vi "UHR-Fleezers Control (host) - 12.7d.vi"() -> ()   [LabVIEW 2012] (continued)
  T22 = cluster{"New Image":T2, "New Image":T2, "New Image":T2, "New Image":T2, "New Image":T2}
  T23 = typedef "XDNodeRunTimeDep.lvlib/timing_clust.ctl" = cluster{"Expected End [f-1]":u64, "Actual End [f-1]":u64, "Finished Late? [f-1]":bool, "Expected End [i-1]":u64, "Actual End [i-1]":u64, "Finished Late? [i-1]":bool, "Expected Start [i]":u64, "Actual Start [i]":u64, "Expected Start [f]":u64, "Actual Start [f]":u64, "Source Name":string, "Structure Name":string, "Period":i64, "Deadline":i64, "Offset":i64, "Start":i64, "Priority":i32, "Timeout":i32, "Mode":T24, "Wakeup Reason":T25, "Error":errorcluster, "Source Type":string, "Secondary Source Type":string, "Global End Time":u64, "Global Start Time":u64, "Frame Duration":u64, "Iteration Duration":u64, "Assigned CPU":i32, "I/O Scan Engine Mode":u32}
  T24 = typedef "XDNodeRunTimeDep.lvlib/nitl_modes.ctl" = enum32{"No Change", "Process missed periods, maintain original phase", "Discard missed periods, maintain original phase", "Process missed periods, ignore original phase", "Discard missed periods, ignore original phase"}
  T25 = typedef "XDNodeRunTimeDep.lvlib/wakeup.ctl" = enum32{"Normal", "Aborted", "Asynchronous wakeup", "Timing source error", "Timed loop error", "Timeout"}
  T26 = enum16{"big-endian, network order", "native, host order", "little-endian"}
  T27 = enum16{"open", "replace", "create", "open or create", "replace or create", "replace or create with confirmation"}
  T28 = cluster{"Scan Range AOD (nm) 2":dbl, "Step Size AOD (nm) 2":dbl, "Scan Speed AOD (nm/s) 2":dbl, "Number of scans (AOD) 2":u16, "Label":string}
  T29 = cluster{"[0]":dbl, "[1]":dbl, "[2]":dbl, "[3]":dbl, "[4]":dbl, "[5]":dbl}
  T30 = cluster{"Diameter (mm)":dbl, "Units":dbl, "Volume":dbl, "Rate":dbl}
  T31 = enum32{"Status", "Sample Stage", "Syringe Pump", "Trap Control (RF)", "APD Counting", "Fluorescence Laser Control", "Trap AI", "Video", "FPGA"}
  T32 = enum32{"Status", "Sample Stage", "Syringe Pump", "Trap Control (RF)", "APD Counting", "Fluorescence Laser Control", "Trap AI", "Video", "FPGA", "Misc. Configuration"}
  T33 = cluster{"Left":i32, "Top":i32, "Width":u32, "Height":u32}
  T34 = cluster{cluster{"Left":i32, "Top":i32, "Width":u32, "Height":u32}}[]
  T35 = enum32{"setting", "request", "request control", "info", "statistics", "system settings", "I/O sub system", "HRT control", "camera descriptions", "device specific data", "event sub system settings", "event sub system results", "image memory manager"}
  T36 = typedef "AviRefnum.ctl" = refnum<k1>
  T37 = typedef "imagedata.ctl" = cluster{"image type":i32, "image depth":i32, "image":u8[], "mask":u8[], "colors":u32[], "Rectangle":cluster{"left":i16, "top":i16, "right":i16, "bottom":i16}}
  T38 = enum32{"Normal Display", "Dual Display (APD)", "FFT", "High Res Display"}
  T39 = cluster{"Origin Pixel":cluster{"X":sgl, "Y":sgl}, "Angle Relative to Horizontal (deg)":sgl, "Axis Reference":u32}
  T40 = typedef "Simple Grid Descriptor" = cluster{"X Step":sgl, "Y Step":sgl, "Unit":T41}
  T41 = typedef "Image Unit" = enum32{"Undefined", "Angström", "Micrometer", "Millimeter", "Centimeter", "Meter", "Kilometer", "Microinch", "Inch", "Feet", "Nautical miles", "Standard miles", "Steps"}
  T42 = cluster{"averaging mode":u16, "weighting mode":u16, "number of averages":u32}
  T43 = cluster{"dB On (F)":bool, "unwrap phase (F)":bool, "convert to degree (F)":bool}
  T44 = cluster{string, string, string, string, string, string, string, string}
  T45 = cluster{string, string, string, string, string, string, string, string, string, string, string, string}
  T46 = cluster{string, string, string, string, string, string, string, string, string, string, string, string, string}
  T47 = cluster{string, string, string, string, string, string, string, string, string, string, string, string, string, string}
  T48 = cluster{"BD 1 Frequency 1 (MHz)":dbl, "BD 1 Frequency 2 (MHz)":dbl}
  T49 = cluster{"f0":dbl, "df":dbl, "magnitude":dbl[]}[][]
  T50 = cluster{"Comment (data description)":string, "Channel 1 Buffer":string, "Channel 2 Buffer":string, "Channel 3 Buffer":string, "Title":string, "DNA Construct":string, "Bead diameter":dbl, "Name":string}
diagram:
  w18 = u16 10 items=["1.0"=10, "1.5"=15, "2.0"=20] ("stop bits (10: 1 bit)")
  w34 = u16 20 items=["1.0"=10, "1.5"=15, "2.0"=20] ("stop bits (10: 1 bit)")
  w37 = u16 20 items=["1.0"=10, "1.5"=15, "2.0"=20] ("stop bits (10: 1 bit)")
  w45 = u16 20 items=["1.0"=10, "1.5"=15, "2.0"=20] ("stop bits (10: 1 bit)")
  w24 = T19 2 items=["Grayscale (U8)", "Grayscale (I16)", "Grayscale (SGL)", "Complex (CSG)", "RGB (U32)", "HSL (U32)", "RGB (U64)", "Grayscale (U16)"] ("Image Type")
  # "Settings to help prevent AOM/D damage"
  # "Initialize the FPGA DAQ card itself"
  # "Reset the DAQ card."
  # "Specify the DAQ card and the FPGA code to run"
  # "Bottom 1 Harvard"
  # "Top 3 Harvard"
  # "Center Harvard"
  # "Bottom 1 Harvard"
  # "Top 3 Harvard"
  # "Center Harvard"
  n1 = case "Trap X limits" shown="\"2axisAOD\"" "1axis AOM vs 2 axis AOD" {
    tunnel: [T16 {"Minimum"=0.0, "Maximum"=40.0, "Increment"=0.1} ("Min Max Inc") T16 {"Minimum"=60.0, "Maximum"=90.0, "Increment"=1.0} ("Min Max Inc")] -> w9
    tunnel: [T16 {"Minimum"=0.0, "Maximum"=45.0, "Increment"=1.0} ("Data Entry Limits") T16 {"Minimum"=0.0, "Maximum"=50.0, "Increment"=1.0} ("Data Entry Limits")] -> w7
    frame "2axisAOD" {
      w81 = u16 300 ("DIO count 1 (ticks)")
      # "Amp Limits"
      # "Freq Limits"
      n2 = disable-structure shown="Disabled" {
        frame Disabled {
          w87 = 35.0 ("BD 1 Amplitude 1 (%)")
          w88 = 30.0 ("BD 1 Frequency 1 (MHz)")
          n3 = local write "BD 1 Frequency 1 (MHz)"(w88) -> ()
          n4 = local write "BD 1 Frequency 2 (MHz)"(w88) -> ()
          n5 = local write "BD 1 Amplitude 2 (%)"(w87) -> ()
          n6 = local write "BD 1 Amplitude 1 (%)"(w87) -> ()
          n7 = local write "BD 2 Frequency 1 (MHz)"(w88) -> ()
          n8 = local write "BD 2 Amplitude 1 (%)"(w87) -> ()
          n9 = local write "BD 2 Frequency 2 (MHz)"(w88) -> ()
          n10 = local write "BD 2 Amplitude 2 (%)"(w87) -> ()
        }
        frame Enabled {
        }
      }
      n11 = local write "All FB On/Off"(FALSE ("All FB On/Off")) -> ()
      n12 = local write "BD 2 Delay (Ticks)"(u8 108 ("BD 2 Delay (Ticks)")) -> ()
      n13 = local write "Number Interlace Sets"(u8 2 ("Number Interlace Sets")) -> ()
      n14 = local write "DIO count 2 (ticks)"(w81) -> ()
      n15 = local write "DIO count 1 (ticks)"(w81) -> ()
    }
    frame "1axis", Default {
      # "Amp Lmits"
      # "Freq Limits"
    }
  }
  n16 = xnode "Open FPGA VI Reference"("resource name"=T18 "750kHzDAQ") -> ("FPGA VI Reference Out"=w14:T20, "error out"=w13:errorcluster)  [unwired: 1 in]
  n17 = xnode "Invoke Method"("FPGA VI Reference In"=w14, "error in"=w13) -> ("FPGA VI Reference Out"=w6:T20, "error out"=→"FPGA error out":errorcluster)
  n18 = flat-sequence "Safety limits on RF frequencies and amplitudes (for AOM protection)" {
    tunnel: [w93] -> w1
    tunnel: [w92] -> w3
    tunnel: [w94] -> w4
    tunnel: [w95] -> w2
    tunnel: w9 -> [w93]
    tunnel: w7 -> [w92]
    tunnel: w6 -> [w91]
    tunnel: [w91] -> w5
    frame #0 {
      w95 = T16 {"Minimum"=0.0, "Maximum"=40.0, "Increment"=0.1} ("Min Max Inc")
      w94 = T16 {"Minimum"=0.0, "Maximum"=45.0, "Increment"=1.0} ("Data Entry Limits")
      n19 = property on="BD 2 Frequency 1 (MHz)" class="DigNum (strict)"("Data Range"=w95) -> ()  [unwired: 2 in, 2 out]
      n20 = property on="BD 2 Frequency 3 (MHz)" class="DigNum (strict)"("Data Range"=w95) -> ()  [unwired: 2 in, 2 out]
      n21 = property on="BD 2 Frequency 2 (MHz)" class="DigNum (strict)"("Data Range"=w95) -> ()  [unwired: 2 in, 2 out]
      n22 = property on="BD 1 Frequency 1 (MHz)" class="DigNum (strict)"("Data Range"=w93) -> ()  [unwired: 2 in, 2 out]
      n23 = property on="BD 1 Frequency 2 (MHz)" class="DigNum (strict)"("Data Range"=w93) -> ()  [unwired: 2 in, 2 out]
      n24 = property on="BD 1 Frequency 3 (MHz)" class="DigNum (strict)"("Data Range"=w93) -> ()  [unwired: 2 in, 2 out]
      n25 = property on="BD 2 Amplitude 1 (%)" class="DigNum (strict)"("Data Range"=w94) -> ()  [unwired: 2 in, 2 out]
      n26 = property on="BD 2 Amplitude 2 (%)" class="DigNum (strict)"("Data Range"=w94) -> ()  [unwired: 2 in, 2 out]
      n27 = property on="BD 2 Amplitude 3 (%)" class="DigNum (strict)"("Data Range"=w94) -> ()  [unwired: 2 in, 2 out]
      n28 = property on="BD 1 Amplitude 3 (%)" class="DigNum (strict)"("Data Range"=w92) -> ()  [unwired: 2 in, 2 out]
      n29 = property on="BD 1 Amplitude 2 (%)" class="DigNum (strict)"("Data Range"=w92) -> ()  [unwired: 2 in, 2 out]
      n30 = property on="BD 1 Amplitude 1 (%)" class="DigNum (strict)"("Data Range"=w92) -> ()  [unwired: 2 in, 2 out]
      "X RF Frequency Limits (MHz)" <- w93
      "X RF Amplitude Limits (%)" <- w92
      "Y RF Amplitude Limits (%)" <- w94
      "Y RF Frequency Limits (MHz)" <- w95
    }
  }
  n31 = stacked-sequence "Host initialization sequence - order matters!" {
    tunnel: w5 -> [_ w98 w196 _ w263 w271 w317 w342 w372]
    tunnel: [_ _ _ _ _ _ _ _ w372] -> w11
    tunnel: [_ _ _ _ _ _ _ _ w371] -> w10
    tunnel: w4 -> [_ _ _ _ _ _ w314 _ _]
    tunnel: w3 -> [_ _ _ _ _ _ w313 _ _]
    tunnel: w2 -> [_ _ _ _ _ _ w312 _ _]
    tunnel: w1 -> [_ _ _ _ _ _ w311 _ _]
    frame #0 {
    }
    frame #1 {
      w131 = 10.0 ("y")
      w132 = 32767.0 ("y")
      w116 = 6.0  # clock mult.
      w115 = 49152000.0  # TCXO frequ.
      # "Initialize some FPGA settings"
      n32 = Build Array("DIO count 1 (ticks)", "DIO count 2 (ticks)", "DIO count 3 (ticks)") -> (w166:u16[])
      n33 = local read "AO1"() -> (w137:dbl)
      n34 = local read "AO2"() -> (w138:dbl)
      n35 = local read "Scan Increment (MHz)"() -> (w120:dbl)
      n36 = property on="AI Count (ticks)" class="DigNum (strict)"("Val(Sgnl)"="AI Count (ticks)") -> ()  [unwired: 2 in, 2 out]
      n37 = local read "Continuous MCL Scanning"() -> (w150:bool)
      n38 = local read "Fast Scan Dir"() -> (w151:bool)
      n39 = local read "Number of scans (MCL)"() -> (w149:u64)
      n40 = Multiply(x=w137, y=w132) -> (x*y=w135:dbl)
      n41 = Multiply(x=w138, y=w132) -> (x*y=w133:dbl)
      n42 = Divide(x=40000000.0, y="AI Count (ticks)") -> (x/y=w155:dbl)
      n43 = Divide(x=w135, y=w131) -> (x/y=w136:dbl)
      n44 = Divide(x=w133, y=w131) -> (x/y=w134:dbl)
      n45 = To Word Integer(number=w136) -> (16bit integer=w139:i16)
      n46 = To Word Integer(number=w134) -> (16bit integer=w140:i16)
      n47 = Not(x=w151) -> (.not. x?=w152:bool)
      n48 = local read "Cycles/step (MCL)"() -> (w148:u64)
      n49 = Multiply(x=w120, y=1000.0) -> (x*y=w113:dbl)
      n50 = local read "Scan steps (MCL)"() -> (w147:u64)
      n51 = local write "Trap Pos FIFO Timeout"(u16 0 ("Trap Pos FIFO Timeout")) -> ()
      n52 = local read "Desired Scan Incr (V)"() -> (w145:dbl)
      n53 = local write "AI rate (Hz)"(w155) -> ()
      n54 = Scale By Power Of 2(n=48, x=w113) -> (x*2^n=w112:dbl)
      n55 = Unbundle By Name(cluster{"output high":i16, "output low":i16} {"output high"=3000, "output low"=0} ("FB output range 1")) -> ("output high"=w185:i16, "output low"=w186:i16)
      n56 = Multiply(x=w115, y=w116) -> (x*y=w117:dbl)
      n57 = Divide(x=w112, y=w117) -> (x/y=w118:dbl)
      n58 = local read "Setpoints (V)"() -> (w105:cluster{"Set 1":dbl, "Set 2":dbl})
      n59 = To Quad Integer(1:w118) -> (0:w121:i64)
      n60 = Multiply(x=w145, y=32767.0) -> (x*y=w143:dbl)
      n61 = Divide(x=w155, y="FPGA Ave.") -> (x/y=w154:dbl)
      n62 = local read "Trap Intensity PID Gains"() -> (w110:T9)
      n63 = local read "Next trap write delay (ticks)"() -> (w189:u8)
      n64 = local read "XY phase ext loop method"() -> (w190:bool)
      n65 = local read "Amp switch delay 2"() -> (w191:u8)
      n66 = local read "BD 2 Delay (Ticks) 2"() -> (w192:u8)
      n67 = local read "BD 1 Delay (ticks) 2"() -> (w193:u8)
      n68 = local write "Ave. Rate (Hz)"(w154) -> ()
      n69 = Reciprocal(x=w154) -> (1/x=w153:dbl)
      n70 = local read "Number Interlace Sets"() -> (w173:u8)
      n71 = Split 1D Array(array=w166, index=w173) -> (first subarray=w164:u16[])  [unwired: 1 out]
      n72 = Add Array Elements(numeric array=w164) -> (sum=w165:u16)
      n73 = local write "Ave. Period (s)"(w153) -> ()
      n74 = local read "# Samples/channel"() -> (w128:u32)
      n75 = local read "Number of F/B Scans (AOD)"() -> (w127:u16)
      n76 = local read "Not-Interlacing Set"() -> (w174:enum32{"Set 1", "Set 2", "Set 3"})
      n77 = To Unsigned Byte Integer(number=w174) -> (unsigned 8bit integer=w168:u8)
      n78 = Index Array(array=w166, index=w168) -> (element=w167:u16)
      n79 = local read "Feedback On/Off"() -> (w102:cluster{"Set 1":bool, "Set 2":bool})
      n80 = local read "BD 2 Delay (Ticks)"() -> (w188:u8)
      n81 = local read "BD 1 Delay (ticks)"() -> (w187:u8)
      n82 = local read "Scan steps (AOD)"() -> (w122:u64)
      n83 = local read "All FB On/Off"() -> (w101:bool)
      n84 = local read "Cycles/step (AOD)"() -> (w123:u64)
      n85 = Divide(x=w143, y=10.0) -> (x/y=w144:dbl)
      n86 = Multiply(x=w122, y=w123) -> (x*y=w124:u64)
      n87 = Unbundle By Name(w110) -> ("proportional gain (Kc)"=w181:i16, "integral gain (Kc*Ts/Ti)"=w182:i16, "derivative gain (Kc*Td/Ts)"=w183:i16)
      n88 = Multiply(x=3276.7, y=w105) -> (x*y=w106:cluster{"Set 1":dbl, "Set 2":dbl})
      n89 = To Word Integer(number=w144) -> (16bit integer=w146:i16)
      n90 = Multiply(x=w124, y=u64 2) -> (x*y=w126:u64)
      n91 = To Word Integer(number=w106) -> (16bit integer=w107:cluster{"Set 1":i16, "Set 2":i16})
      n92 = Multiply(x=w126, y=w127) -> (x*y=w129:u64)
      n93 = local read "Sets to FIFO (Traps)"() -> (w177:T15)
      n94 = Divide(x=w129, y=w128) -> (x/y=w130:dbl)
      n95 = Unbundle By Name(w107) -> ("Set 1"=w108:i16, "Set 2"=w109:i16)
      n96 = local read "2D or 1D Scan"() -> (w163:bool)
      n97 = local write "Data points/scans"(w129) -> ()
      n98 = local read "Scan BD"() -> (w111:bool)
      n99 = And(x=w102, y=w101) -> (x .and. y?=w103:cluster{"Set 1":bool, "Set 2":bool})
      n100 = local write "Data points/scan (f/b)"(w126) -> ()
      n101 = local read "N Acq Sets (Traps + Fl.)"() -> (w159:i16)
      n102 = local write "N sets should be saved"(w130) -> ()
      n103 = local read "FPGA error out"() -> (w97:errorcluster)
      n104 = Unbundle By Name(w103) -> ("Set 1"=w99:bool, "Set 2"=w100:bool)
      n105 = local read "Interlace"() -> (w172:bool)
      n106 = Select(t=w165, s=w172, f=w167) -> (s? t:f=w175:u16)
      n107 = local write "Update Count (MCL)"(w175) -> ()
      n108 = local write "Total Counts (ticks)"(w175) -> ()
      n109 = Unbundle By Name(w177) -> ("Set 1"=w178:bool, "Set 2"=w179:bool, "Set 3"=w180:bool)
      n110 = property on="2D or 1D Scan" class="Bool (strict)"("Val(Sgnl)"=w163) -> ()  [unwired: 2 in, 2 out]
      n111 = xnode "Read/Write Control"("FPGA VI Reference In"=w98, "error in"=w97, "ai count"="AI Count (ticks)", "Interlace ON/OFF"=w172, "Number Interlace Cycles"=w173, "Set 1"=w178, "Set 2"=w179, "Set 3"=w180, "FB On/Off Set 1"=w99, "FB On/Off Set 2"=w100, "Interlace Off Parameters"=w174, "FB Setpoint Set 1"=w108, "FB Setpoint Set 2"=w109, "P1"=w181, "I1"=w182, "D1"=w183, "FB1 output high"=w185, "FB1 output low"=w186, "Cycles per step"=w123, "Scan BD"=w111, "Number of scans"=w127, "Scan steps"=w122, "Scan freq.  increment"=w121, "AO1"=w139, "AO2"=w140, "Scan freq.  increment (MCL)"=w146, "Scan steps (MCL)"=w147, "Cycles per step (MCL)"=w148, "Number of scans (MCL)"=w149, "MCL count"=w175, "Cont. Scan (MCL)"=w150, "MCL Scan Axis"=w152, "1D or 2D Scan?"=w163, "N of AI1 Int Acq Sets"=w159, "Amp switch delay"="Amp switch delay", "Swap F1 and F2"="Swap F1 and F2", "APD to FIFO"=FALSE, "DIO count 1 (ticks)"="DIO count 1 (ticks)", "DIO count 2 (ticks)"="DIO count 2 (ticks)", "DIO count 3 (ticks)"="DIO count 3 (ticks)", "BD 1 Delay (ticks)"=w187, "BD 2 Delay (Ticks)"=w188, "Next trap write delay (ticks)"=w189, "XY phase ext loop method"=w190, "Amp switch delay 2"=w191, "BD 2 Delay (Ticks) 2"=w192, "BD 1 Delay (ticks) 2"=w193) -> ("error out"=w96:errorcluster)  [unwired: 1 in, 1 out]
      n112 = local write "FPGA error out"(w96) -> ()
    }
    frame #2 {
      # "Initialize some more FPGA settings"
      n113 = local read "Laser interlacing mode"() -> (w197:enum32{"Laser ON", "Laser OFF", "Interlace"})
      n114 = local read "Green Laser ON"() -> (w198:bool)
      n115 = local read "Trap Pos. FB Range"() -> (w220:T12)
      n116 = local read "Trap Pos. FB Gains"() -> (w221:T11)
      n117 = Multiply(x="Green Intensity % (FB OFF)", y=655.35) -> (x*y=w203:dbl)
      n118 = local read "Invert laser interlacing"() -> (w240:bool)
      n119 = local read "Trap Pos. AI1 X Pre-scale"() -> (w214:u16)
      n120 = Multiply(x="Green FB Setpoint (mV)", y=3.2767) -> (x*y=w206:dbl)
      n121 = local read "Trap Pos FB Int Count"() -> (w216:u16)
      n122 = local read "Differential FB?"() -> (w219:bool)
      n123 = local read "Neg. TTrig FPGA"() -> (w217:bool)
      n124 = Multiply(x="Red FB Setpoint (mV)", y=3.2767) -> (x*y=w232:dbl)
      n125 = To Unsigned Word Integer(number=w203) -> (unsigned 16bit integer=w205:u16)
      n126 = Multiply(x="Red Intensity % (FB OFF)", y=655.35) -> (x*y=w236:dbl)
      n127 = To Word Integer(number=w206) -> (16bit integer=w208:i16)
      n128 = Unbundle By Name("Green FB Gains") -> ("proportional gain (Kc)"=w229:i16, "integral gain (Kc*Ts/Ti)"=w230:i16, "derivative gain (Kc*Td/Ts)"=w231:i16)
      n129 = Unbundle By Name("Red FB Gains") -> ("proportional gain (Kc)"=w243:i16, "integral gain (Kc*Ts/Ti)"=w244:i16, "derivative gain (Kc*Td/Ts)"=w245:i16)
      n130 = case shown="False" w198 {
        tunnel: w197 -> [_ w248]
        tunnel: [enum32{"Laser ON", "Laser OFF", "Interlace"}."Laser OFF" ("Green laser mode") w248] -> w241
        frame False {
        }
        frame True {
        }
      }
      n131 = To Word Integer(number=w232) -> (16bit integer=w235:i16)
      n132 = Unbundle By Name(w221) -> ("proportional gain (Kc)"=w225:fxp<+/-,16,8>, "integral gain (Kc*Ts/Ti)"=w226:fxp<+/-,16,8>, "derivative gain (Kc*Td/Ts)"=w227:fxp<+/-,16,8>)
      n133 = To Unsigned Word Integer(number=w236) -> (unsigned 16bit integer=w239:u16)
      n134 = Unbundle By Name(w220) -> ("output high"=w222:fxp<+/-,16,1>, "output low"=w224:fxp<+/-,16,1>)
      n135 = local read "Trap Pos FB Monitor\nT1 or T2"() -> (w209:bool)
      n136 = local read "Trap Pos FB Negate Action"() -> (w210:bool)
      n137 = local read "Trap Pos. FB Offset Factor"() -> (w211:i64)
      n138 = local read "Trap Pos. FB Mult Factor"() -> (w212:i64)
      n139 = local read "FPGA error out"() -> (w194:errorcluster)
      n140 = xnode "Read/Write Control"("FPGA VI Reference In"=w196, "error in"=w194, "Invert GI 2"=w240, "Operating Mode 2"=w241, "P3"=w229, "I3"=w230, "D3"=w231, "Green FB Setpoint"=w208, "Green FB On/Off"="Green FB On/Off", "Current Out"=w205, "Green int current ON count adj"="Green int current ON count adj", "Operating Mode"=w241, "Invert GI"=w240, "Trap Pos FB Monitor T1 or T2"=w209, "Trap Pos FB Negate Action"=w210, "Trap Pos. FB Offset Factor"=w211, "Trap Pos. FB Mult Factor"=w212, "Force feedback"=FALSE, "AI1 X Scale"=w214, "Trap Pos to FIFO"=TRUE, "Trap Pos FB Int Count"=w216, "TTrig Negate Pos"=w217, "FB Trig Integrate"="FB Trig Integrate", "Diff FB Measurement?"=w219, "Negate Diff?"="Negate Diff?", "P2"=w225, "I2"=w226, "D2"=w227, "FB2 output high"=w222, "FB2 output low"=w224, "Red FB Setpoint"=w235, "RI Current Out"=w239, "Red Laser Operating Mode"=w241, "RI Operating Mode 2"=w241, "Invert RI 2"=w240, "Invert RI"=w240, "P4"=w243, "I4"=w244, "D4"=w245, "Red FB On/Off"="Red FB On/Off") -> ("error out"=w195:errorcluster)  [unwired: 1 out]
      n141 = local write "FPGA error out"(w195) -> ()
    }
    frame #3 {
      # "Initialize more settings. Should stop using event loops to initialize."
      # "What are these?"
      n142 = stacked-sequence {
        frame #0 {
          w251 = T21."empty" ("mode")
          # "Clear external fluorescence triggering FIFO"
          # "APD loop counts"
          # "Fluorescence loop counts (rates)"
          n143 = local read "APD Integration Time (s)"() -> (w253:dbl)
          n144 = local read "Interlace ON count"() -> (w254:u16)
          n145 = call "Smart Buffer (DBL) 1.vi"("mode"=w251) -> ()  [unwired: 5 in, 6 out]
          n146 = call "Smart Buffer (DBL) 2.vi"("mode"=w251) -> ()  [unwired: 5 in, 6 out]
          n147 = property on="APD Integration Time (s)" class="DigNum (strict)"("Val(Sgnl)"=w253) -> ()  [unwired: 2 in, 2 out]
          n148 = property on="Interlace ON count" class="DigNum (strict)"("Val(Sgnl)"=w254) -> ()  [unwired: 2 in, 2 out]
          "Number of APDs" <- 3.0 ("Number of APDs")
        }
        frame #1 {
          # "Number of APDs affects\nAPD DMA transfer"
          # "General settings for all lasers:"
          # "And includes all laser\nON/OFF settings"
          # "Fluorescent lasers settings:"
          # "Blue laser settings:"
          n149 = local read "Laser interlacing mode"() -> (w256:enum32{"Laser ON", "Laser OFF", "Interlace"})
          n150 = local read "Invert laser interlacing"() -> (w255:bool)
          n151 = local read "Blue FB On/Off"() -> (w257:bool)
          n152 = property on="Blue FB On/Off" class="Bool (strict)"("Val(Sgnl)"=w257) -> ()  [unwired: 2 in, 2 out]
          n153 = property on="Invert laser interlacing" class="Bool (strict)"("Val(Sgnl)"=w255) -> ()  [unwired: 2 in, 2 out]
          n154 = property on="Laser interlacing mode" class="RadioBtnsControl (strict)"("Val(Sgnl)"=w256) -> ()  [unwired: 2 in, 2 out]
        }
        frame #2 {
          w258 = path "C:/Home/wheeler/Comstock-LabView-Link.udl" ("connection information")
          # "Initialize the database connection"
          n155 = call-poly <vilib>:"DB Tools Open Connection.vi"("connection information"=w258) -> ("connection reference"=w259:T17)  [unwired: 7 in, 1 out]
          "connection reference" <- w259
          n156 = local write "connection reference"(w259) -> ()
          n157 = local write "Database link"(w258) -> ()
        }
        frame #3 {
          n158 = Wait (ms)(milliseconds to wait=u32 5000) -> ()  [unwired: 1 out]
        }
      }
      n159 = local write "Offset (nm)"(0.0 ("Offset (nm)")) -> ()
      n160 = local write "Bead Mean (nm)"(0.0 ("Bead Mean (nm)")) -> ()
    }
    frame #4 {
      # "Set FIFO size and run FPGA"
      n161 = local read "FPGA error out"() -> (w262:errorcluster)
      n162 = xnode "Invoke Method"("FPGA VI Reference In"=w263, "error in"=w262, "Requested Depth"="Trap AI FIFO Depth") -> ("FPGA VI Reference Out"=w267:T20, "error out"=w268:errorcluster)  [unwired: 1 out]
      n163 = xnode "Invoke Method"("FPGA VI Reference In"=w267, "error in"=w268, "Requested Depth"="Trap Position FIFO Depth") -> ("FPGA VI Reference Out"=w265:T20, "error out"=w264:errorcluster)  [unwired: 1 out]
      n164 = xnode "Invoke Method"("FPGA VI Reference In"=w265, "error in"=w264) -> ("error out"=w261:errorcluster)  [unwired: 1 in, 1 out]
      n165 = local write "FPGA error out"(w261) -> ()
    }
    frame #5 {
      # "Adjust FPGA timing loop phases"
      n166 = flat-sequence "Initial FPGA Loop Relative Phase Adjustment" {
        tunnel: "Initial Phase Adjustment (AI1)" -> [w302]
        tunnel: "Initial Phase Adjustment (GI)" -> [w301]
        tunnel: "Initial Phase Adj. (MCL)" -> [w300]
        tunnel: [w303] -> w287
        tunnel: [w299] -> w286
        tunnel: "Initial Phase Adjustment (APD Acq)" -> [w298]
        tunnel: "Initial Phase Adjustment (APD 1 Gate)" -> [w297]
        tunnel: "Initial Phase Adjustment (Green FB)" -> [w296]
        tunnel: "Initial Phase Adjustment (GI) 2" -> [w295]
        tunnel: "Initial Phase Adjustment (APD 2 Gate)" -> [w294]
        tunnel: "Initial Phase Adjustment (RI)" -> [w293]
        tunnel: "Initial Phase Adjustment (BI DO)" -> [w292]
        tunnel: "Initial Phase Adjustment (BI AO)" -> [w291]
        tunnel: "Initial Phase Adjustment (APD 3 Gate)" -> [w290]
        tunnel: w271 -> [w289]
        tunnel: w287 -> [w305]
        tunnel: [w306] -> w285
        tunnel: w286 -> [w306]
        tunnel: [w305] -> w284
        tunnel: w285 -> [w310]
        tunnel: w284 -> [w309]
        tunnel: [w307] -> w270
        frame #0 {
          n167 = local read "FPGA error out"() -> (w288:errorcluster)
          n168 = xnode "Read/Write Control"("FPGA VI Reference In"=w289, "error in"=w288, "Phase count adjustment"=w302, "Phase count adjustment (GI)"=w301, "Phase count adjustment (MCL)"=w300, "Phase Count Adjustment (APD Acq)"=w298, "Phase count adjustment (APD 1 Gate)"=w297, "Phase count adjustment (APD 2 Gate)"=w294, "Phase count adjustment (Green FB)"=w296, "Phase count adjustment (GI) 2"=w295, "Phase count adjustment (RI)"=w293, "Phase count adjustment (BI AO)"=w291, "Phase count adjustment (BI D)"=w292, "Phase count adjustment (APD 3 Gate)"=w290) -> ("FPGA VI Reference Out"=w299:T20, "error out"=w303:errorcluster)
        }
        frame #1 {
          n169 = Wait (ms)(milliseconds to wait=u32 100) -> ()  [unwired: 1 out]
        }
        frame #2 {
          w308 = TRUE
          n170 = xnode "Read/Write Control"("FPGA VI Reference In"=w310, "error in"=w309, "+ phase"=w308, "+ phase (GI)"=w308, "+ phase (MCL)"=w308, "+ phase (APD Acq)"=w308, "+ phase (APD 1 Gate)"=w308, "+ phase (APD 2 Gate)"=w308, "+ phase (Green FB)"=w308, "+ phase (GI) 2"=w308, "+ phase (RI)"=w308, "+ phase (BI AO)"=w308, "+ phase (BI D)"=w308, "+ phase (APD 3 Gate)"=w308) -> ("error out"=w307:errorcluster)  [unwired: 1 out]
        }
      }
      n171 = local write "FPGA error out"(w270) -> ()
    }
    frame #6 {
      # "Initialize trap RF synth board and set initial frequencies and amplitudes"
      n172 = local read "FPGA error out"() -> (w316:errorcluster)
      n173 = call "Initialize RF boards - interlace 3.vi"("error in"=w316, "FPGA VI Reference In"=w317) -> ("error out"=w318:errorcluster, "FPGA VI Reference Out"=w339:T20)
      n174 = call "set RF board frequency - interlace.vi"("Board 2 Frequency Limits"=w312, "Board 1 Frequency Limits"=w311, "error in"=w318, "FPGA VI Reference In"=w339, "Board 2 Frequency 3 (MHz)"="BD 2 Frequency 3 (MHz)", "Board 1 Frequency 3 (MHz)"="BD 1 Frequency 3 (MHz)", "Board 2 Frequency 2 (MHz)"="BD 2 Frequency 2 (MHz)", "Board 2 Frequency 1 (MHz)"="BD 2 Frequency 1 (MHz)", "Board 1 Frequency 2 (MHz)"="BD 1 Frequency 2 (MHz)", "Board 1 Frequency 1  (MHz)"="BD 1 Frequency 1 (MHz)") -> ("error out"=w322:errorcluster, "FPGA VI Reference Out"=w321:T20)
      n175 = call "set RF board amplitude - interlace.vi"("Board 2 Amplitude Limits"=w314, "Board 1 Amplitude Limits"=w313, "error in"=w322, "FPGA VI Reference In"=w321, "Board 2 Amplitude 3 (%)"="BD 2 Amplitude 3 (%)", "Board 1 Amplitude 3 (%)"="BD 1 Amplitude 3 (%)", "Board 2 Amplitude 2 (%)"="BD 2 Amplitude 2 (%)", "Board 2 Amplitude 1 (%)"="BD 2 Amplitude 1 (%)", "Board 1 Amplitude 2 (%)"="BD 1 Amplitude 2 (%)", "Board 1 Amplitude 1 (%)"="BD 1 Amplitude 1 (%)") -> ("error out"=w315:errorcluster)  [unwired: 1 out]
      n176 = Subtract(x="BD 1 Frequency 1 (MHz)", y="BD 1 Frequency 2 (MHz)") -> (x-y=w329:dbl)
      n177 = Subtract(x="BD 2 Frequency 1 (MHz)", y="BD 2 Frequency 2 (MHz)") -> (x-y=w330:dbl)
      n178 = local write "FPGA error out"(w315) -> ()
      n179 = Square(x=w330) -> (x^2=w332:dbl)
      n180 = Square(x=w329) -> (x^2=w331:dbl)
      n181 = Add(x=w331, y=w332) -> (x+y=w333:dbl)
      n182 = Square Root(x=w333) -> (sqrt(x)=w334:dbl)
      n183 = local write "Trap Delta (MHz)"(w334) -> ()
    }
    frame #7 {
      n184 = local read "FPGA error out"() -> (w341:errorcluster)
      n185 = flat-sequence {
        tunnel: [w356] -> w346
        tunnel: [w355] -> w345
        tunnel: w342 -> [w348]
        tunnel: w341 -> [w347]
        tunnel: [w360] -> w344
        tunnel: w346 -> [w360]
        tunnel: [w359] -> w343
        tunnel: w345 -> [w359]
        tunnel: w344 -> [w368]
        tunnel: w343 -> [w367]
        tunnel: [w362] -> w340
        frame #0 {
          w349 = FALSE ("Retract Pump 3")
          n186 = local read "Trap 1 (ON/OFF)"() -> (w350:bool)
          n187 = xnode "Read/Write Control"("FPGA VI Reference In"=w348, "error in"=w347, "Direct RF Box  Communication"=FALSE) -> ("FPGA VI Reference Out"=w356:T20, "error out"=w355:errorcluster)
          n188 = local write "Saving..."(FALSE ("Saving Data")) -> ()
          n189 = local write "Stop All"(FALSE ("Stop All")) -> ()
          n190 = local write "Retract Pump 1"(w349) -> ()
          n191 = local write "Retract Pump 3"(w349) -> ()
          n192 = local write "Index"(1.0 ("Index")) -> ()
          n193 = property on="Trap 1 ON" class="Bool (strict)"("Value"=w350) -> ()  [unwired: 2 in, 2 out]
          "Manipulating Trap" <- FALSE ("Manipulating Trap")
        }
        frame #1 {
          n194 = local read "Trap 2 (ON/OFF)"() -> (w358:bool)
          n195 = Wait (ms)(milliseconds to wait=u32 10) -> ()  [unwired: 1 out]
          n196 = property on="Trap 2 ON" class="Bool (strict)"("Val(Sgnl)"=w358) -> ()  [unwired: 2 in, 2 out]
        }
        frame #2 {
          n197 = local read "Scan Range (nm)"() -> (w363:dbl)
          n198 = xnode "Read/Write Control"("FPGA VI Reference In"=w368, "error in"=w367, "FPGA Controls  RF Box"=TRUE ("Direct RF Box  Communication")) -> ("error out"=w362:errorcluster)  [unwired: 1 out]
          n199 = call "Update messages.vi"("Message to add"="UHR-Fleezers ready.", "Old message string"="") -> ("New message string"=w366:string)
          n200 = local write "Messages"(w366) -> ()
          n201 = property on="Scan Range (nm)" class="DigNum (strict)"("Val(Sgnl)"=w363) -> ()  [unwired: 2 in, 2 out]
        }
      }
      n202 = local write "FPGA error out"(w340) -> ()
    }
    frame #8 {
      # "Wait 5 s for all the event loops still being executed to finish."
      n203 = Wait (ms)(milliseconds to wait=u32 5000) -> ()  [unwired: 1 out]
      n204 = local read "FPGA error out"() -> (w371:errorcluster)
    }
  }
  n205 = call-poly "VISA Configure Serial Port"("VISA resource name"="VISA resource name", "baud rate (9600)"=u32 115200, "stop bits (10: 1 bit)"=w18) -> ("VISA resource name out"=w17:refnum<visa-resource-name>, "error out"=w16:errorcluster)  [unwired: 4 in, 7 out]
  n206 = call-poly "VISA Configure Serial Port"("VISA resource name"="Bottom  1 Harvard Syringe Pump Serial Port", "baud rate (9600)"=u32 115200, "stop bits (10: 1 bit)"=w34) -> ("VISA resource name out"=w30:refnum<visa-resource-name>, "error out"=w29:errorcluster)  [unwired: 4 in, 7 out]
  n207 = call-poly "VISA Configure Serial Port"("VISA resource name"="Top 3 Harvard Syringe Pump Serial Port", "baud rate (9600)"=u32 115200, "stop bits (10: 1 bit)"=w37) -> ("VISA resource name out"=w32:refnum<visa-resource-name>, "error out"=w31:errorcluster)  [unwired: 4 in, 7 out]
  n208 = call-poly "VISA Configure Serial Port"("VISA resource name"="Sample Chamber Stage Serial Port") -> ("VISA resource name out"=w58:refnum<visa-resource-name>, "error out"=w59:errorcluster)  [unwired: 5 in, 8 out]
  "Stage Control Serial Error" <- w59
  n209 = local write "Blue Error Out"(w16) -> ()
  n210 = call-poly "VISA Configure Serial Port"("VISA resource name"="Center Harvard Syringe Pump Serial Port", "baud rate (9600)"=u32 115200, "stop bits (10: 1 bit)"=w45) -> ("VISA resource name out"=w42:refnum<visa-resource-name>, "error out"=w43:errorcluster)  [unwired: 4 in, 7 out]
  n211 = call "IMAQ Create"("Image Name"="APD 1 Image", "Image Type"=w24) -> ("New Image"=w51:T2)  [unwired: 3 in, 1 out]
  n212 = call "IMAQ Create"("Image Name"="APD 2 Image", "Image Type"=w24) -> ("New Image"=w50:T2)  [unwired: 3 in, 1 out]
  n213 = call "IMAQ Create"("Image Name"="APD 3 Image", "Image Type"=w24) -> ("New Image"=w23:T2)  [unwired: 3 in, 1 out]
  n214 = call "IMAQ Create"("Image Name"="Det. X Image", "Image Type"=w24) -> ("New Image"=w49:T2)  [unwired: 3 in, 1 out]
  n215 = call "IMAQ Create"("Image Name"="Det. Y Image", "Image Type"=w24) -> ("New Image"=w48:T2)  [unwired: 3 in, 1 out]
  n216 = Bundle("New Image"=w51, "New Image"=w50, "New Image"=w23, "New Image"=w49, "New Image"=w48) -> (w47:T22)  [unwired: 1 in]
  n217 = node-c288(2 ("Processor")) -> (w66:T23)  [unwired: 3 out]
  n218 = node-c288() -> (w22:T23)  [unwired: 4 out]
  n219 = node-c288() -> (w54:T23)  [unwired: 4 in]
  n220 = node-c288(3 ("Processor")) -> (w64:T23)  [unwired: 3 out]
  n221 = node-c288() -> (w68:T23)  [unwired: 4 out]
  n222 = while "Duncan's play event loop" {
    stop <- w374 stop-if-true
    n223 = Create User Event(user event datatype=TRUE ("Boolean")) -> (user event=w375:refnum<user-event>)  [unwired: 1 in, 1 out]
    n224 = Create User Event(user event datatype=TRUE ("Boolean")) -> (user event=w382:refnum<user-event>)  [unwired: 1 in, 1 out]
    n225 = global write "Global for fluorescence simulation mean (30 samples), (power series).vi" "Red Signal"(w375) -> ()
    n226 = global write "Global for fluorescence simulation mean (30 samples), (power series).vi" "Green Signal"(w382) -> ()
    n227 = register-events(w382, w375) -> (reference out=w381:refnum<event-registration>)  [unwired: 2 in, 1 out]
    n228 = event shown="[1] \"Get Fluorophore\": Value Change" {
      selector: w381 -> [_ _ _ _]
      dyn-events: _ -> [_ _ _ _]
      timeout: 100 -> [_ _ _ _]
      event Timeout {
        n229 = event-data() -> ()  [unwired: 1 in, 2 out]
      }
      event "Get Fluorophore": Value Change {
        n230 = event-data() -> ("OldVal"=w384:bool)  [unwired: 1 in, 4 out]
        n231 = case shown="True" w384 {
          selector: w384 -> [_ w385]
          frame False {
          }
          frame True {
            n232 = property on="Move to Position 3" class="Bool"("Val(Sgnl)"=w385) -> ()  [unwired: 2 in, 2 out]
            n233 = case shown="1" "Numeric" {
              frame 0, Default {
              }
              frame 1 {
                n234 = property on="Green Laser ON" class="Bool (strict)"("Val(Sgnl)"=TRUE ("Value (Signaling)")) -> ()  [unwired: 2 in, 2 out]
              }
              frame 2 {
                n235 = property on="Red Laser ON" class="Bool (strict)"("Val(Sgnl)"=TRUE) -> ()  [unwired: 2 in, 2 out]
              }
            }
          }
        }
      }
      event User Event {
        n236 = event-data() -> ("Boolean"=w389:bool)  [unwired: 1 in, 3 out]
        "Green Fluorophore" <- w389
        n237 = property on="Get Fluorophore" class="Bool (strict)"("Val(Sgnl)"=w389) -> ()  [unwired: 2 in, 2 out]
      }
      event User Event {
        n238 = event-data() -> ("Boolean"=w390:bool)  [unwired: 1 in, 3 out]
        "Red Fluorophore" <- w390
        n239 = property on="Get Fluorophore" class="Bool (strict)"("Val(Sgnl)"=w390) -> ()  [unwired: 2 in, 2 out]
      }
    }
    n240 = property on="Get Fluorophore" class="Bool (strict)"("Val(Sgnl)"="Get Fluorophore") -> ()  [unwired: 2 in, 2 out]
    n241 = Wait (ms)(milliseconds to wait=u32 100) -> ()  [unwired: 1 out]
    n242 = local read "Stop All"() -> (w373:bool)
    n243 = Or(x=w373, y="stop") -> (x .or. y?=w374:bool)
  }
  n244 = timed-loop "Basic control parameters (all FPGA settings, other basic controls)" {
    shift-right: [w398] -> _
    shift-left: errorcluster {"status"=FALSE, "code"=0, "source"=""} ("error out") -> [_]
    tunnel: [w397] -> _
    timing: w66 -> [_]
    timing-out: [_] -> w65
    tunnel: w42 -> [w396]
    tunnel: w32 -> [w395]
    tunnel: w31 -> [w394]
    tunnel: w30 -> [w393]
    tunnel: w29 -> [w392]
    tunnel: w5 -> [w391]
    stop <- w397 stop-if-true
    n245 = node-c288() -> ()  [unwired: 2 out]
    n246 = event shown="[66] \"Remove Unwinding Offset\": Value Change" {
      selector: _ -> [_ _ _ _ _ _ _ _ _ _ _ _ _ _ _ _ _ _ _ _ _ _ _ _ _ _ _ _ _ _ _ _ _ _ _ _ _ _ _ _ _ _ _ _ _ _ _ _ _ _ _ _ _ _ _ _ _ _ _ _ _ _ _ _ _ _ _ _ _ _ _ _ _ _]
      dyn-events: _ -> [_ _ _ _ _ _ _ _ _ _ _ _ _ _ _ _ _ _ _ _ _ _ _ _ _ _ _ _ _ _ _ _ _ _ _ _ _ _ _ _ _ _ _ _ _ _ _ _ _ _ _ _ _ _ _ _ _ _ _ _ _ _ _ _ _ _ _ _ _ _ _ _ _ _]
      timeout: _ -> [_ _ _ _ _ _ _ _ _ _ _ _ _ _ _ _ _ _ _ _ _ _ _ _ _ _ _ _ _ _ _ _ _ _ _ _ _ _ _ _ _ _ _ _ _ _ _ _ _ _ _ _ _ _ _ _ _ _ _ _ _ _ _ _ _ _ _ _ _ _ _ _ _ _]
      tunnel: [w438 _ _ _ w467 _ _ _ _ _ _ w538 _ _ w606 w608 w617 w619 w689 _ w708 w732 w752 w772 w791 w815 w844 _ w849 w943 w947 w984 _ w1018 w1021 w1024 w1034 w1037 _ w1044 _ _ _ _ _ _ _ _ _ _ _ _ _ _ _ _ _ w1421 _ _ _ _ w1457 _ _ _ _ _ _ _ _ _ _ _] -> w398
      tunnel: [_ _ _ _ _ _ _ _ _ w523 _ _ _ _ _ _ _ _ _ _ _ _ _ _ _ _ _ _ _ _ _ _ _ _ _ _ _ _ _ _ _ _ _ _ _ _ _ _ _ _ _ _ _ _ _ _ _ _ _ _ _ _ _ _ _ _ _ _ _ _ _ _ _ _] -> w397
      tunnel: [_ _ _ _ _ _ _ "Round T1 X" _ _ _ _ _ _ _ _ _ _ _ _ _ _ _ _ _ _ _ _ _ _ _ _ _ _ _ _ _ _ _ _ _ _ _ _ _ _ _ _ _ _ _ _ _ _ _ _ _ _ _ _ _ _ _ _ _ _ _ _ _ _ _ _ _ _] -> _
      tunnel: [_ _ _ "Adjust Scale\nto Mean" _ _ _ _ _ _ _ _ _ _ _ _ _ _ _ _ _ _ _ _ _ _ _ _ "Test ttrig" _ _ _ _ _ _ _ _ _ _ _ _ _ _ _ _ _ _ "Flush Sample" "Flush Pump 3" "Flush Pump 1" "Clear Volume" _ _ _ _ _ _ _ _ _ _ _ _ _ _ _ _ _ _ _ _ _ _ _] -> _
      tunnel: [_ _ _ _ _ _ _ _ "Round T2 X" _ "Delayed Interlace Start" _ _ _ _ _ _ _ _ _ _ _ _ _ _ _ _ _ _ _ _ _ _ _ _ _ _ _ _ _ _ _ _ _ _ _ _ _ _ _ _ _ _ _ _ _ _ _ _ _ _ _ _ _ _ _ _ _ _ _ _ _ _ _] -> _
      tunnel: w396 -> [_ _ _ _ _ _ _ _ _ _ _ _ _ _ _ _ _ _ _ _ _ _ _ _ _ _ _ _ _ _ _ _ _ _ _ _ _ _ _ _ _ _ _ w1201 w1208 w1215 w1220 w1229 _ _ w1335 _ _ _ _ _ _ _ _ _ _ _ _ _ _ _ _ _ _ _ _ _ _ _]
      tunnel: w395 -> [_ _ _ _ _ _ _ _ _ _ _ _ _ _ _ _ _ _ _ _ _ _ _ _ _ _ _ _ _ _ _ _ _ _ _ _ _ _ _ _ _ w1118 _ _ _ _ _ _ w1273 _ _ w1341 _ w1350 _ w1364 _ _ _ _ _ _ _ _ _ _ _ _ _ _ _ _ _ _]
      tunnel: w394 -> [_ _ _ _ _ _ _ _ _ _ _ _ _ _ _ _ _ _ _ _ _ _ _ _ _ _ _ _ _ _ _ _ _ _ _ _ _ _ _ _ _ _ _ _ _ _ _ _ _ _ _ _ _ _ _ _ _ _ _ _ _ _ _ _ _ _ _ _ _ _ _ _ _ _]
      tunnel: w393 -> [_ _ _ _ _ _ _ _ _ _ _ _ _ _ _ _ _ _ _ _ _ _ _ _ _ _ _ _ _ _ _ _ _ _ _ _ _ _ _ _ w1055 _ _ _ _ _ _ _ _ w1303 _ _ w1346 _ w1357 _ w1389 _ _ _ _ _ _ _ _ _ _ _ _ _ _ _ _ _]
      tunnel: w392 -> [_ _ _ _ _ _ _ _ _ _ _ _ _ _ _ _ _ _ _ _ _ _ _ _ _ _ _ _ _ _ _ _ _ _ _ _ _ _ _ _ _ _ _ _ _ _ _ _ _ _ _ _ _ _ _ _ _ _ _ _ _ _ _ _ _ _ _ _ _ _ _ _ _ _]
      tunnel: w391 -> [w401 _ _ _ w466 _ w492 _ _ _ _ w529 _ _ w584 w607 w612 w618 w654 _ w697 w730 w733 w753 w773 w792 w820 w845 w847 w851 w944 w948 _ w1015 w1019 w1022 w1032 w1035 _ w1043 _ _ _ _ _ _ _ _ _ _ _ _ _ _ _ _ _ w1414 _ w1435 _ w1441 w1456 _ w1463 w1465 w1472 w1486 w1501 _ w1510 _ w1530 _]
      event "AI Count (ticks)", "Sets to FIFO (Traps)", "Save ave N", "FPGA Ave.", "# Samples/channel", "N sets to save": Value Change {
        # "So that if 'Save ave N' is updated, the AOD scanning code updates too."
        n247 = event-data() -> ()  [unwired: 6 out]
        n248 = local read "AI Count (ticks)"() -> (w422:u16)
        n249 = Unbundle By Name("Sets to FIFO (Traps)") -> ("Set 1"=w405:bool, "Set 2"=w404:bool, "Set 3"=w403:bool)
        n250 = Boolean To (0,1)(Boolean="Sets to FIFO (Traps)") -> (0, 1=w430:cluster{"Set 1":i16, "Set 2":i16, "Set 3":i16})
        n251 = xnode "Read/Write Control"("FPGA VI Reference In"=w401, "ai count"=w422, "Set 1"=w405, "Set 2"=w404, "Set 3"=w403, "N of AI1 Int Acq Sets"="N Acq Sets (Traps + Fl.)") -> ("error out"=w438:errorcluster)  [unwired: 1 in, 1 out]
        n252 = Cluster To Array(cluster=w430) -> (array=w429:i16[])
        n253 = To Unsigned Long Integer(number=w429) -> (unsigned 32bit integer=w411:u32[])
        n254 = local read "Scan steps (AOD)"() -> (w431:u64)
        n255 = Multiply(x=w422, y="N Acq Sets (Traps + Fl.)") -> (x*y=w420:u16)
        n256 = Divide(x=40000000.0, y=w422) -> (x/y=w414:dbl)
        "AI rate (Hz)" <- w414
        "Ave. Rate (Hz)" <- w414
        n257 = Add Array Elements(numeric array=w411) -> (sum=w423:u32)
        "Trap Sets" <- w423
        n258 = Reciprocal(x=w414) -> (1/x=→"Ave. Period (s)":dbl)
        n259 = property on="Scan steps (AOD)" class="DigNum (strict)"("Val(Sgnl)"=w431) -> ()  [unwired: 2 in, 2 out]
        n260 = Divide(x=w414, y="N Acq Sets (Traps + Fl.)") -> (x/y=w435:dbl)
        "Data Rate (Hz)" <- w435
        n261 = Reciprocal(x=w435) -> (1/x=→"Data Period (s)":dbl)
        n262 = local read "Save ave N"() -> (w434:dbl)
        n263 = Divide(x=w435, y=w434) -> (x/y=w433:dbl)
        "Save Data Rate (Hz)" <- w433
        n264 = Reciprocal(x=w433) -> (1/x=→"Save Data Period (s)":dbl)
        n265 = Multiply(x=w420, y="# Samples/trap") -> (x*y=w418:u32)
        "Counts/DMA" <- w418
        n266 = property on="Trap Disp. Downsample" class="DigNum (strict)"("Maximum"="# Samples/trap") -> ()  [unwired: 2 in, 2 out]
        n267 = Multiply(x=w423, y="# Samples/trap") -> (x*y=w412:u32)
        "# Samples/channel" <- w412
        n268 = Multiply(x=w412, y=u32 8) -> (x*y=→"Trap AI Elements/DMA read":u32)
        n269 = local read "APD Int. Count"() -> (w419:u32)
        n270 = Multiply(x=w412, y=u32 3) -> (x*y=→"Trap Pos Elements/DMA read":u32)
        n271 = Divide(x=w418, y=w419) -> (x/y=w409:dbl)
        "APD Samples/FIFO Acq." <- w409
        n272 = Divide(x=w418, y=40000000.0) -> (x/y=w416:dbl)
        "DMA Update Period (s)" <- w416
        n273 = local read "Number of APDs"() -> (w402:u8)
        n274 = Multiply(x=w402, y=w409) -> (x*y=→"APD Elements/DMA read":dbl)
        n275 = property on="APD Disp. Downsample" class="DigNum (strict)"("Maximum"=w409) -> ()  [unwired: 2 in, 2 out]
        n276 = local read "N sets to save"() -> (w428:u32)
        n277 = Multiply(x=w416, y=w428) -> (x*y=→"Total Time (s)":dbl)
        "FPGA Averaging" <- FALSE ("FPGA Averaging")
      }
      event "Remove Offset": Value Change {
        n278 = event-data() -> ()  [unwired: 7 out]
        n279 = local write "Remove Offset"(FALSE ("Remove Offset")) -> ()
        n280 = local read "Bead Mean (nm)"() -> (w440:dbl)
        n281 = local read "Offset (nm)"() -> (w441:dbl)
        n282 = Add(x=w440, y=w441) -> (x+y=w439:dbl)
        n283 = local write "Offset (nm)"(w439) -> ()
        n284 = disable-structure shown="Disabled" {
          frame Disabled {
            n285 = local read "Bead Mean (nm)"() -> (w446:dbl)
            n286 = Add(y=w446) -> (x=w445:dbl, x+y=w444:dbl)
            n287 = Subtract(x=w446, y=w445) -> (x-y=w443:dbl)
            n288 = property on="Bead Separation" class="WFChart (strict)"("YScale.Minimum"=w443) -> ()  [unwired: 2 in, 2 out]
            n289 = property on="Bead Separation" class="WFChart (strict)"("YScale.Maximum"=w444) -> ()  [unwired: 2 in, 2 out]
          }
          frame Enabled {
          }
        }
      }
      event "Detector Type": Value Change {
        n290 = event-data() -> ()  [unwired: 7 out]
        n291 = local read "AI labels"() -> (w447:string[])
        n292 = property on="High Res. Display" class="Ring (strict)"("Strings []"=w447) -> ()  [unwired: 2 in, 2 out]
        n293 = Build Array (concatenate)(w447, "none") -> (w448:string[])
        n294 = property on="FFT 1 Choice 1" class="Ring (strict)"("Strings []"=w448) -> ()  [unwired: 2 in, 2 out]
        n295 = property on="FFT 1 Choice 2" class="Ring (strict)"("Strings []"=w448) -> ()  [unwired: 2 in, 2 out]
        n296 = property on="FFT 2 Choice 1" class="Ring (strict)"("Strings []"=w448) -> ()  [unwired: 2 in, 2 out]
        n297 = property on="FFT 2 Choice 2" class="Ring (strict)"("Strings []"=w448) -> ()  [unwired: 2 in, 2 out]
        n298 = Bundle("APD 1", "APD 2") -> (w451:cluster{string, string})  [unwired: 1 out]
        n299 = Cluster To Array(cluster=w451) -> (array=w449:string[])
        n300 = Build Array (concatenate)(w449, w448) -> (w453:string[])
        n301 = Array Size(array=w453) -> (size(s)=w454:i32)
        n302 = property on="Signals to Plot" class="LstBox (strict)"("Item Names"=w453) -> ()  [unwired: 2 in, 2 out]
        n303 = property on="Signals to Plot" class="LstBox (strict)"("Number of Rows"=w454) -> ()  [unwired: 2 in, 2 out]
        n304 = property on="All Signals" class="WFChart (strict)"("LegNumRows"=w454) -> ()  [unwired: 2 in, 2 out]
      }
      event "Adjust Scale\nto Mean": Value Change {
        n305 = event-data() -> ()  [unwired: 7 out]
        n306 = local read "APD 1 Rate (Hz)"() -> (w463:dbl)
        n307 = Multiply(x=1000.0, y="Above (kHz)") -> (x*y=w461:dbl)
        n308 = Multiply(x=1000.0, y="Below (kHz)") -> (x*y=w459:dbl)
        n309 = Add(x=w461, y=w463) -> (x+y=w456:dbl)
        n310 = Subtract(x=w463, y=w459) -> (x-y=w457:dbl)
        n311 = property on="APD Chart" class="WFChart (strict)"("YScale.Minimum"=w457) -> ()  [unwired: 2 in, 2 out]
        n312 = property on="APD Chart" class="WFChart (strict)"("YScale.Maximum"=w456) -> ()  [unwired: 2 in, 2 out]
      }
      event "Phase adj. (AI1)", "+ phase (AI1)", "- phase (AI1)": Value Change {
        n313 = event-data() -> ()  [unwired: 7 out]
        n314 = Negate(x="Phase adj. (AI1)") -> (-x=w474:i16)
        n315 = Select(t=w474, s="- phase (AI1)", f="Phase adj. (AI1)") -> (s? t:f=w473:i16)
        n316 = xnode "Read/Write Control"("FPGA VI Reference In"=w466, "Phase count adjustment"=w473) -> ("FPGA VI Reference Out"=w472:T20, "error out"=w471:errorcluster)  [unwired: 2 in]
        n317 = Or(x="- phase (AI1)", y="+ phase (AI1)") -> (x .or. y?=w468:bool)
        n318 = xnode "Read/Write Control"("FPGA VI Reference In"=w472, "error in"=w471, "+ phase"=w468) -> ("error out"=w467:errorcluster)  [unwired: 1 in, 1 out]
      }
      event "Signals to Plot": Double Click {
        w478 = u32 9868950 ("Color Box")
        n319 = event-data() -> ("Row"=w480:i32)  [unwired: 9 out]
        n320 = property on="All Signals" class="WFChart (strict)"("Active Plot"=w480) -> (error out=w491:errorcluster)  [unwired: 2 in, 1 out]
        n321 = property on="All Signals" class="WFChart (strict)" props=["Plot", "Visible?", "Plot", "Plot Color"](error in=w491) -> (error out=w490:errorcluster, "Plot.Visible?"=w489:bool)  [unwired: 1 in, 2 out]
        n322 = Select(t=FALSE ("Plot.Visible"), s=w489, f=TRUE ("Plot.Visible")) -> (s? t:f=w484:bool)
        n323 = property on="All Signals" class="WFChart (strict)"(error in=w490, "Plot.Visible?"=w484) -> (error out=w486:errorcluster)  [unwired: 1 in, 1 out]
        n324 = property on="All Signals" class="WFChart (strict)"(error in=w486) -> (error out=w481:errorcluster, "Plot.Plot Color"=w485:u32)  [unwired: 1 in, 1 out]
        n325 = property on="Signals to Plot" class="LstBox (strict)"(error in=w481, "Active Row"=w480) -> (error out=w479:errorcluster)  [unwired: 1 in, 1 out]
        n326 = Select(t=w485, s=w484, f=u32 0) -> (s? t:f=w482:u32)
        n327 = property on="Signals to Plot" class="LstBox (strict)"(error in=w479, "CellFontColor"=w482, "SelColor"=w478, "CellBG"=w478, "CellFontSize"=u32 20 ("Active Row:Cell Font:Size"), "CellFontBold"=TRUE ("Active Row:Cell Font:Bold")) -> ()  [unwired: 1 in, 2 out]
      }
      event "BD 1 Frequency 1 (MHz)", "BD 1 Frequency 2 (MHz)", "BD 1 Frequency 3 (MHz)", "BD 2 Frequency 1 (MHz)", "BD 2 Frequency 2 (MHz)", "BD 2 Frequency 3 (MHz)", "Trap Delta (MHz)", "Update all trap values": Value Change {
        # "This is so you can set trap frequencies\nvia local variables and then update\nall at once"
        n328 = event-data() -> ("CtlRef"=w496:refnum<vi>)  [unwired: 6 out]
        n329 = control-ref of="Trap Delta (MHz)"() -> (w495:refnum<vi>)
        n330 = Equal?(x=w495, y=w496) -> (x = y?=w494:bool)
        n331 = local write "Update all trap values"(FALSE ("Update all trap values")) -> ()
        n332 = case shown="False" "Oscillate Set 1" {
          tunnel: w494 -> [w500 _]
          tunnel: w492 -> [w498 _]
          frame False {
            n333 = local read "BD 1 Frequency 2 (MHz)"() -> (w504:dbl)
            n334 = local read "BD 1 Frequency 1 (MHz)"() -> (w502:dbl)
            n335 = Subtract(x=w504, y="Trap Delta (MHz)") -> (x-y=w501:dbl)
            n336 = Select(t=w501, s=w500, f=w502) -> (s? t:f=w499:dbl)
            n337 = local read "Y RF Frequency Limits (MHz)"() -> (w505:T16)
            n338 = local read "X RF Frequency Limits (MHz)"() -> (w506:T16)
            n339 = local write "BD 1 Frequency 1 (MHz)"(w499) -> ()
            n340 = local read "BD 1 Frequency 3 (MHz)"() -> (w515:dbl)
            n341 = local read "BD 2 Frequency 1 (MHz)"() -> (w509:dbl)
            n342 = local read "BD 2 Frequency 2 (MHz)"() -> (w508:dbl)
            n343 = local read "BD 2 Frequency 3 (MHz)"() -> (w516:dbl)
            n344 = call "set RF board frequency - interlace.vi"("Board 2 Frequency Limits"=w505, "Board 1 Frequency Limits"=w506, "FPGA VI Reference In"=w498, "Board 2 Frequency 3 (MHz)"=w516, "Board 1 Frequency 3 (MHz)"=w515, "Board 2 Frequency 2 (MHz)"=w508, "Board 2 Frequency 1 (MHz)"=w509, "Board 1 Frequency 2 (MHz)"=w504, "Board 1 Frequency 1  (MHz)"=w499) -> ()  [unwired: 1 in, 2 out]
            n345 = Subtract(x=w509, y=w508) -> (x-y=w513:dbl)
            n346 = Subtract(x=w499, y=w504) -> (x-y=w514:dbl)
            n347 = Square(x=w513) -> (x^2=w511:dbl)
            n348 = Square(x=w514) -> (x^2=w512:dbl)
            n349 = Add(x=w512, y=w511) -> (x+y=w510:dbl)
            n350 = Square Root(x=w510) -> (sqrt(x)=w507:dbl)
            n351 = property on="Initial delta (MHz)" class="DigNum (strict)"("Val(Sgnl)"=w507) -> ()  [unwired: 2 in, 2 out]
            n352 = local write "Trap Delta (MHz)"(w507) -> ()
          }
          frame True {
          }
        }
      }
      event "Round T1 X": Value Change {
        n353 = event-data() -> ()  [unwired: 7 out]
        n354 = local read "BD 1 Frequency 1 (MHz)"() -> (w519:dbl)
        n355 = Round To Nearest(number=w519) -> (nearest integer value=w518:dbl)
        n356 = property on="BD 1 Frequency 1 (MHz)" class="DigNum (strict)"("Val(Sgnl)"=w518) -> ()  [unwired: 2 in, 2 out]
      }
      event "Round T2 X": Value Change {
        n357 = event-data() -> ()  [unwired: 7 out]
        n358 = local read "BD 1 Frequency 2 (MHz)"() -> (w521:dbl)
        n359 = Round To Nearest(number=w521) -> (nearest integer value=w520:dbl)
        n360 = property on="BD 1 Frequency 2 (MHz)" class="DigNum (strict)"("Val(Sgnl)"=w520) -> ()  [unwired: 2 in, 2 out]
      }
      event "Stop All": Value Change {
        n361 = event-data() -> ()  [unwired: 7 out]
        n362 = local read "Stop All"() -> (w523:bool)
      }
      event "Delayed Interlace Start": Value Change {
        n363 = event-data() -> ()  [unwired: 7 out]
        n364 = flat-sequence {
          frame #0 {
            n365 = Multiply(x="Delay to Interlace (s)", y=1000.0) -> (x*y=w525:dbl)
            n366 = Wait (ms)(milliseconds to wait=w525) -> ()  [unwired: 1 out]
          }
          frame #1 {
            n367 = property on="Laser interlacing mode" class="RadioBtnsControl (strict)"("Val(Sgnl)"=enum32{"Laser ON", "Laser OFF", "Interlace"}."Interlace" ("Value (Signaling)")) -> ()  [unwired: 2 in, 2 out]
          }
        }
      }
      event "BD 1 Amplitude 1 (%)", "BD 1 Amplitude 2 (%)", "BD 1 Amplitude 3 (%)", "BD 2 Amplitude 1 (%)", "BD 2 Amplitude 2 (%)", "BD 2 Amplitude 3 (%)", "Trap 1 ON", "Trap 2 ON", "Trap 3 ON", "Feedback On/Off", "All FB On/Off": Value Change {
        w550 = i16 1 ("f")
        n368 = event-data() -> ()  [unwired: 7 out]
        n369 = local write "Trap 1 (ON/OFF)"("Trap 1 ON") -> ()
        n370 = local write "Trap 2 (ON/OFF)"("Trap 2 ON") -> ()
        n371 = Boolean To (0,1)(Boolean="Trap 3 ON") -> (0, 1=w551:i16)
        n372 = Boolean To (0,1)(Boolean="Trap 1 ON") -> (0, 1=w552:i16)
        n373 = Boolean To (0,1)(Boolean="Trap 2 ON") -> (0, 1=w553:i16)
        n374 = Select(t=w553, s="Trap ON/OFF X or Y Amp?", f=w550) -> (s? t:f=w548:i16)
        n375 = Select(t=w552, s="Trap ON/OFF X or Y Amp?", f=w550) -> (s? t:f=w549:i16)
        n376 = Select(t=w551, s="Trap ON/OFF X or Y Amp?", f=w550) -> (s? t:f=w547:i16)
        n377 = Select(t=w550, s="Trap ON/OFF X or Y Amp?", f=w553) -> (s? t:f=w545:i16)
        n378 = Select(t=w550, s="Trap ON/OFF X or Y Amp?", f=w552) -> (s? t:f=w546:i16)
        n379 = Select(t=w550, s="Trap ON/OFF X or Y Amp?", f=w551) -> (s? t:f=w544:i16)
        n380 = And(x="All FB On/Off", y="Feedback On/Off") -> (x .and. y?=w542:cluster{"Set 1":bool, "Set 2":bool})
        n381 = local read "BD 1 Amplitude 1 (%)"() -> (w560:dbl)
        n382 = local read "BD 1 Amplitude 2 (%)"() -> (w559:dbl)
        n383 = local read "BD 1 Amplitude 3 (%)"() -> (w558:dbl)
        n384 = Unbundle By Name(w542) -> ("Set 1"=w537:bool, "Set 2"=w534:bool)
        n385 = local read "Y RF Amplitude Limits (%)"() -> (w530:T16)
        n386 = local read "X RF Amplitude Limits (%)"() -> (w531:T16)
        n387 = local read "BD 2 Amplitude 1 (%)"() -> (w561:dbl)
        n388 = local read "BD 2 Amplitude 2 (%)"() -> (w562:dbl)
        n389 = local read "BD 2 Amplitude 3 (%)"() -> (w563:dbl)
        n390 = And(x="Trap 2 ON", y=w534) -> (x .and. y?=w532:bool)
        n391 = And(x="Trap 1 ON", y=w537) -> (x .and. y?=w535:bool)
        n392 = Multiply(x=w549, y=w560) -> (x*y=w557:dbl)
        n393 = Multiply(x=w559, y=w548) -> (x*y=w555:dbl)
        n394 = Multiply(x=w558, y=w547) -> (x*y=w556:dbl)
        n395 = Multiply(x=w561, y=w546) -> (x*y=w564:dbl)
        n396 = Multiply(x=w562, y=w545) -> (x*y=w565:dbl)
        n397 = Multiply(x=w563, y=w544) -> (x*y=w566:dbl)
        n398 = call "set RF board amplitude - interlace.vi"("Board 2 Amplitude Limits"=w530, "Board 1 Amplitude Limits"=w531, "FPGA VI Reference In"=w529, "Board 2 Amplitude 3 (%)"=w566, "Board 1 Amplitude 3 (%)"=w556, "Board 2 Amplitude 2 (%)"=w565, "Board 2 Amplitude 1 (%)"=w564, "Board 1 Amplitude 2 (%)"=w555, "Board 1 Amplitude 1 (%)"=w557) -> ("error out"=w539:errorcluster, "FPGA VI Reference Out"=w540:T20)  [unwired: 1 in]
        n399 = xnode "Read/Write Control"("FPGA VI Reference In"=w540, "error in"=w539, "FB On/Off Set 1"=w535, "FB On/Off Set 2"=w532) -> ("error out"=w538:errorcluster)  [unwired: 1 out]